vi "Initialise.vi"(6 "Font":T1=enum."Starcon", 8 "error in (no error)":errorcluster, 11 "Renderer":u32) -> (0 "error out":errorcluster, 3 "Font out":refnum<class "Sprite Font.lvclass">)   [LabVIEW 2021, in "Sprite Font.lvclass"]
uses:
  Sprite Font.lvclass
  Re-use Libraries/Vector 2D/Vector 2D.lvclass
  Sprite Font.lvclass/Sprite Font.ctl
  Resource Manager/Resource Manager.lvclass
  Character.ctl
  Game Font.ctl
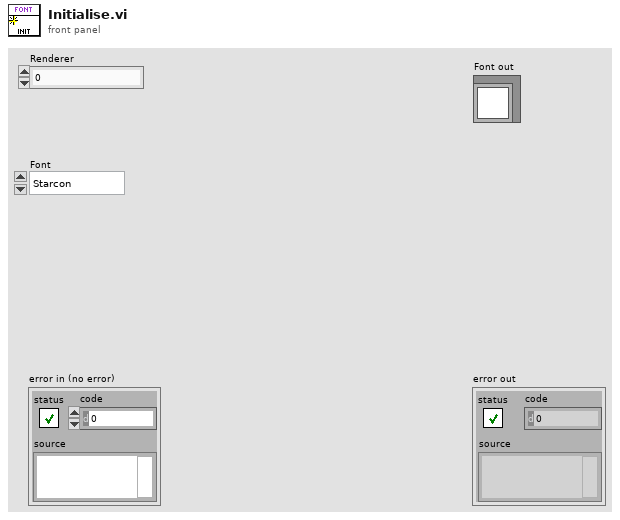
[diagram p1: front panel]
types:
  T1 = typedef "Sprite Font.lvclass/Game Font.ctl" = enum16{"Ilwrath", "Micro", "Slylandro", "Starcon", "Tiny", "Utwig"}
  T2 = typedef "Sprite Font.lvclass/Character.ctl" = cluster{"Texture Name":string, "Size":refnum<class "Vector 2D.lvclass">}
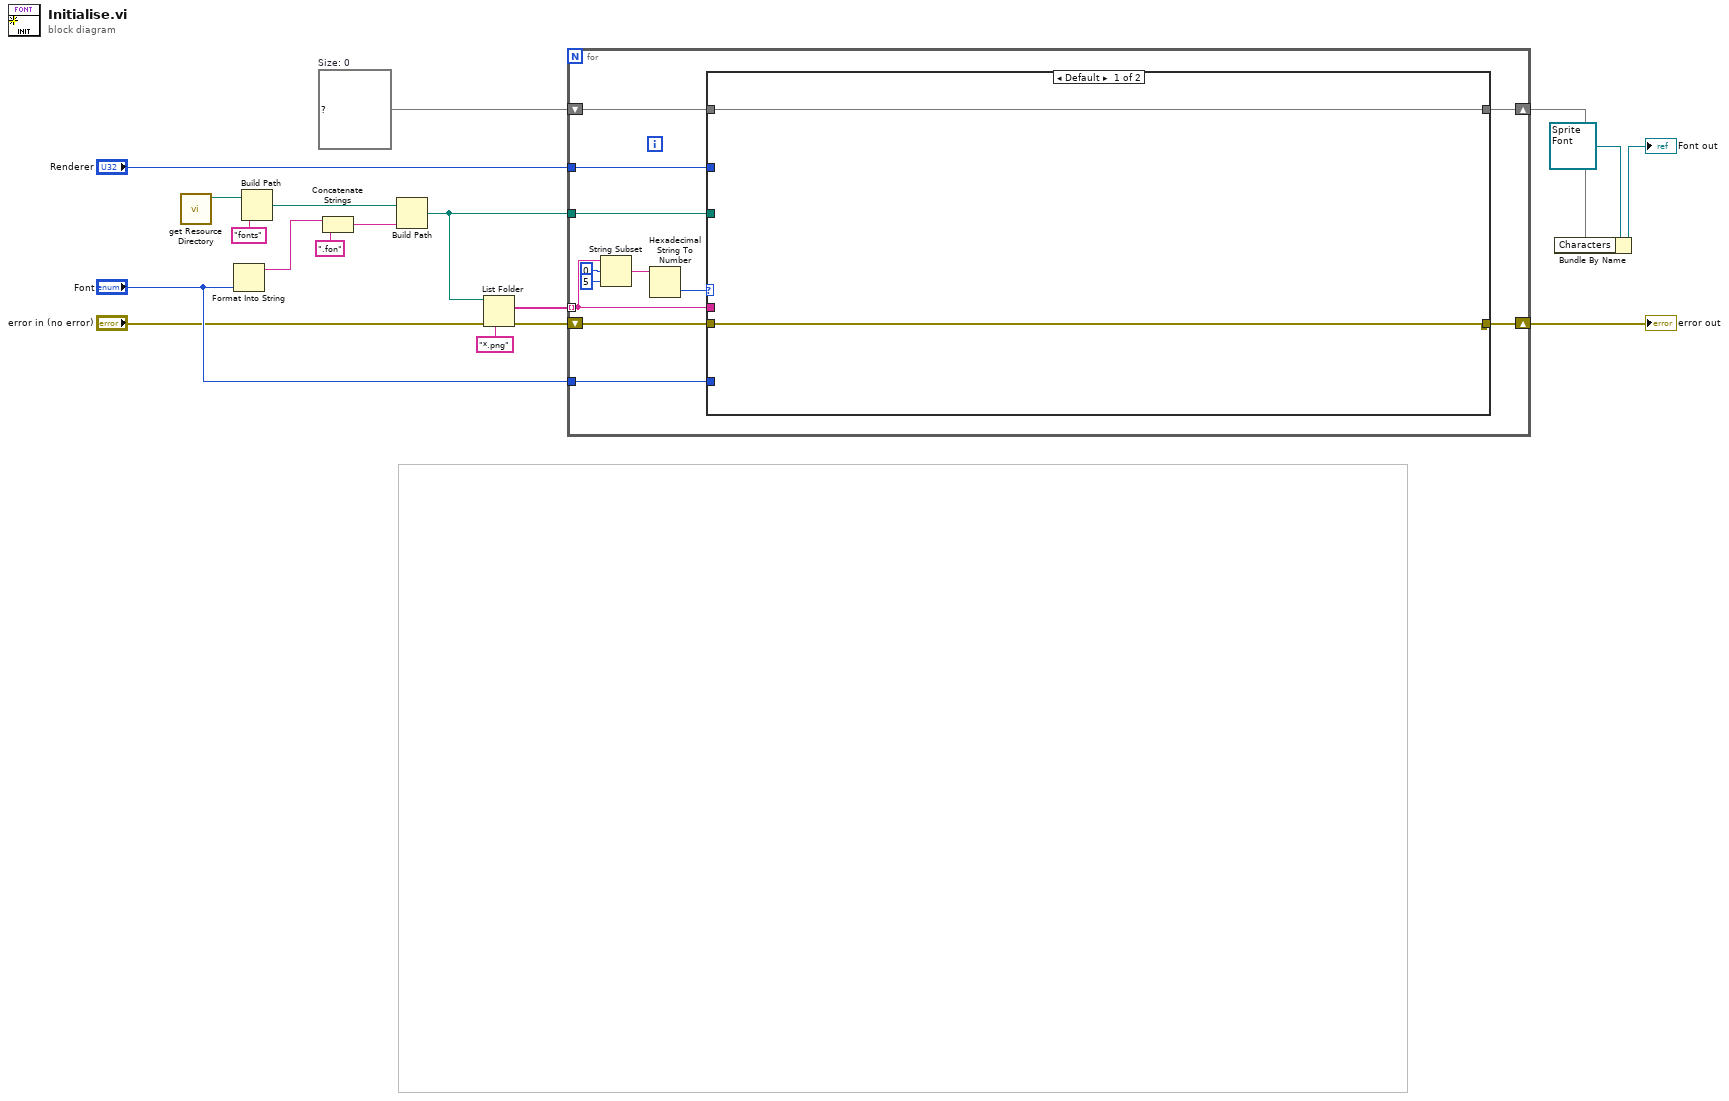
[diagram p0: block diagram]
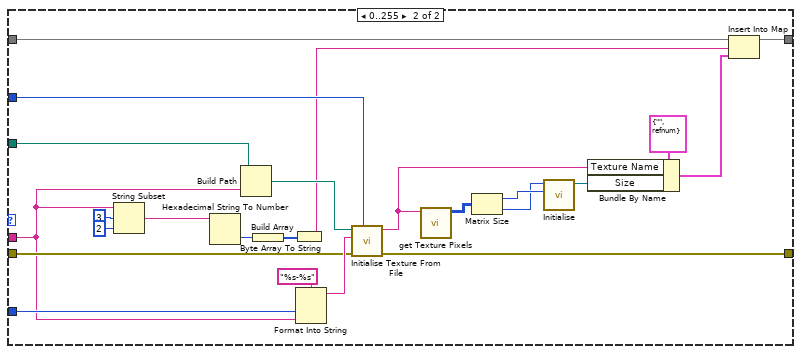
[diagram p2: hidden frame]
diagram:
  w8 = map{string, T2} {}  # Size: 0
  n1 = call "get Resource Directory.vi"() -> ("Resource Directory"=w18:path)  [unwired: 11 in]
  n2 = Format Into String("Font") -> (resulting string=w6:string)  [unwired: 3 in, 1 out]
  n3 = Build Path(base path=w18, name or relative path="fonts") -> (appended path=w16:path)
  n4 = Concatenate Strings(w6, ".fon" ("string")) -> (w9:string)
  n5 = Build Path(base path=w16, name or relative path=w9) -> (appended path=w3:path)
  n6 = List Folder(path=w3, pattern="*.png", error in="error in (no error)") -> (filenames=w1:string[], error out=w4:errorcluster)  [unwired: 1 in, 2 out]
  n7 = for {
    tunnel: "Renderer" -> [w30]
    tunnel: "Font" -> [w29]
    shift-right: [w28] -> w13
    shift-left: w4 -> [w24]
    tunnel: w3 -> [w27]
    shift-right: [w25] -> w7
    shift-left: w8 -> [w26]
    tunnel: w1 -> [w19] mode=indexing
    n8 = String Subset(string=w19, offset (0)=0, length (rest)=5 ("length (rest)")) -> (substring=w21:string)
    n9 = Hexadecimal String To Number(string=w21) -> (number=w20:u32)  [unwired: 2 in, 1 out]
    n10 = case shown="Default" w20 {
      tunnel: w30 -> [_ w56]
      tunnel: w29 -> [_ w54]
      tunnel: [w31 w52] -> w28
      tunnel: w27 -> [_ w50]
      tunnel: w26 -> [w32 w43]
      tunnel: [w32 w42] -> w25
      tunnel: w24 -> [w31 w40]
      tunnel: w19 -> [_ w39]
      frame Default {
      }
      frame 0..255 {
        n11 = String Subset(string=w39, offset (0)=3, length (rest)=2 ("length (rest)")) -> (substring=w36:string)
        n12 = Hexadecimal String To Number(string=w36) -> (number=w35:u32)  [unwired: 2 in, 1 out]
        n13 = Build Path(base path=w50, name or relative path=w39) -> (appended path=w51:path)
        n14 = Build Array(w35) -> (w34:u32[])
        n15 = Byte Array To String(unsigned byte array=w34) -> (string=w33:string)
        n16 = Format Into String(format string="%s-%s", w54, w39) -> (resulting string=w53:string)  [unwired: 2 in, 1 out]
        n17 = call "Initialise Texture From File.vi"("Renderer"=w56, "error in (no error)"=w40, "Name"=w53, "File"=w51) -> ("error out"=w52:errorcluster, "Name In Cache"=w47:string)  [unwired: 6 in]
        n18 = call "get Texture Pixels.vi"("Texture Name"=w47) -> ("Pixels"=w49:u32[][])  [unwired: 10 in]
        n19 = Matrix Size(0:w49) -> (1:w46:i32, 2:w45:i32)
        n20 = call "Initialise.vi"("y"=w46, "x"=w45) -> ("Vector 2D out"=w44:refnum<class "Vector 2D.lvclass">)  [unwired: 9 in]
        n21 = Bundle By Name(cluster=T2 {"Texture Name"="", "Size"=refnum} ("Character"), "Texture Name"=w47, "Size"=w44) -> (w41:T2)
        n22 = Insert Into Map(map in=w43, key=w33, value=w41) -> (map out=w42:map{string, T2})  [unwired: 2 out]
      }
    }
  }
  "error out" <- w13
  n23 = Bundle By Name(cluster=refnum<class "Sprite Font.lvclass"> refnum ("Galaxy in"), "Characters"=w7) -> (→"Font out":refnum<class "Sprite Font.lvclass">)
